vi "FlexMag - 23-03-2023.vi"() -> ()   [LabVIEW 2018] (continued)
                            tunnel: [w16037 TRUE ("CH1_Trns_BP_Left_DO")] -> w16029
                            frame False {
                              n10680 = local read "CH2_TGV_Control_DI"() -> (w16038:bool)
                              n10681 = case shown="False" w16038 {
                                tunnel: [FALSE ("CH1_Trns_BP_Left_DO") TRUE ("CH1_Trns_BP_Left_DO")] -> w16037
                                frame False {
                                n10682 = Wait Until Next ms Multiple(millisecond multiple=u32 200) -> ()  [unwired: 1 out]
                                n10683 = local write "CH2_TGV_Control_DO"(TRUE ("CH1_Trns_BP_Left_DO")) -> ()
                                }
                                frame True {
                                }
                              }
                            }
                            frame True {
                            }
                          }
                          n10684 = local read "ch2-1 transfer"() -> (w16036:bool)
                          n10685 = local read "ABORT"() -> (w16035:bool)
                          n10686 = Not(x=w16036) -> (.not. x?=w16034:bool)
                          n10687 = Compound Arithmetic op=OR(w16029, w16035, w16034) -> (w16033:bool)
                        }
                      }
                      frame True {
                      }
                    }
                  }
                }
              }
              frame #12 {
                n10688 = local read "ch2-1 transfer"() -> (w16046:bool)
                n10689 = case shown="True" w16046 {
                  frame False {
                  }
                  frame True {
                    n10690 = local read "ABORT"() -> (w16047:bool)
                    n10691 = case shown="False" w16047 {
                      frame False {
                        w16048 = TRUE ("CH2_Right_Limit_DO")
                        n10692 = local write "trns 2-1 led 5"(TRUE ("trns 1-2 led 1")) -> ()
                        n10693 = Wait (ms)(milliseconds to wait=u32 100) -> ()  [unwired: 1 out]
                        n10694 = local write "CH2_Right_Limit_DO"(w16048) -> ()
                        n10695 = local write "CH2_Right_Slow_DO"(w16048) -> ()
                        n10696 = local write "CH2_Left_Slow_DO"(w16048) -> ()
                        n10697 = local write "CH2_Left_Limit_DO"(w16048) -> ()
                      }
                      frame True {
                      }
                    }
                  }
                }
              }
              frame #13 {
                n10698 = local read "ch2-1 transfer"() -> (w16051:bool)
                n10699 = case shown="True" w16051 {
                  frame False {
                  }
                  frame True {
                    n10700 = local read "ABORT"() -> (w16052:bool)
                    n10701 = case shown="False" w16052 {
                      frame False {
                        n10702 = while {
                          i -> [w16057]
                          stop <- w16058 stop-if-true
                          n10703 = local read "CH3_Trns_Interlock_DI"() -> (w16053:bool)
                          n10704 = Greater Or Equal?(x=w16057, y=100) -> (x >= y?=w16055:bool)
                          n10705 = case shown="True" w16055 {
                            frame False {
                            }
                            frame True {
                              n10706 = local write "Warning Message"("Transfer process canceled!\nCH3 Interlock problem" ("Warning Message")) -> ()
                              n10707 = local write "trns error"(TRUE ("TRNS error")) -> ()
                            }
                          }
                          n10708 = case shown="False" w16053 {
                            tunnel: [w16062 TRUE ("CH1_Trns_BP_Left_DO")] -> w16054
                            frame False {
                              n10709 = local read "CH3_TGV_Control_DI"() -> (w16063:bool)
                              n10710 = case shown="False" w16063 {
                                tunnel: [FALSE ("CH1_Trns_BP_Left_DO") TRUE ("CH1_Trns_BP_Left_DO")] -> w16062
                                frame False {
                                n10711 = Wait Until Next ms Multiple(millisecond multiple=u32 200) -> ()  [unwired: 1 out]
                                n10712 = local write "CH3_TGV_Control_DO"(TRUE ("CH1_Trns_BP_Left_DO")) -> ()
                                }
                                frame True {
                                }
                              }
                            }
                            frame True {
                            }
                          }
                          n10713 = local read "ch2-1 transfer"() -> (w16061:bool)
                          n10714 = local read "ABORT"() -> (w16060:bool)
                          n10715 = Not(x=w16061) -> (.not. x?=w16059:bool)
                          n10716 = Compound Arithmetic op=OR(w16054, w16060, w16059) -> (w16058:bool)
                        }
                      }
                      frame True {
                      }
                    }
                  }
                }
              }
              frame #14 {
                n10717 = local read "ch2-1 transfer"() -> (w16071:bool)
                n10718 = case shown="True" w16071 {
                  frame False {
                  }
                  frame True {
                    n10719 = local read "ABORT"() -> (w16072:bool)
                    n10720 = case shown="False" w16072 {
                      frame False {
                        n10721 = local write "trns 2-1 led 6"(TRUE ("trns 1-2 led 1")) -> ()
                        n10722 = Wait (ms)(milliseconds to wait=u32 100) -> ()  [unwired: 1 out]
                      }
                      frame True {
                      }
                    }
                  }
                }
              }
              frame #15 {
                n10723 = local read "ch2-1 transfer"() -> (w16075:bool)
                n10724 = case shown="True" w16075 {
                  frame False {
                  }
                  frame True {
                    n10725 = local read "ABORT"() -> (w16076:bool)
                    n10726 = case shown="False" w16076 {
                      frame False {
                        n10727 = while {
                          i -> [w16081]
                          stop <- w16082 stop-if-true
                          n10728 = local read "CH4_Trns_Interlock_DI"() -> (w16077:bool)
                          n10729 = Greater Or Equal?(x=w16081, y=100) -> (x >= y?=w16079:bool)
                          n10730 = case shown="True" w16079 {
                            frame False {
                            }
                            frame True {
                              n10731 = local write "Warning Message"("Transfer process canceled!\nCH4 Interlock problem" ("Warning Message")) -> ()
                              n10732 = local write "trns error"(TRUE ("TRNS error")) -> ()
                            }
                          }
                          n10733 = case shown="False" w16077 {
                            tunnel: [w16086 TRUE ("CH1_Trns_BP_Left_DO")] -> w16078
                            frame False {
                              n10734 = local read "CH4_TGV_Control_DI"() -> (w16087:bool)
                              n10735 = case shown="False" w16087 {
                                tunnel: [FALSE ("CH1_Trns_BP_Left_DO") TRUE ("CH1_Trns_BP_Left_DO")] -> w16086
                                frame False {
                                n10736 = Wait Until Next ms Multiple(millisecond multiple=u32 200) -> ()  [unwired: 1 out]
                                n10737 = local write "CH4_TGV_Control_DO"(TRUE ("CH1_Trns_BP_Left_DO")) -> ()
                                }
                                frame True {
                                }
                              }
                            }
                            frame True {
                            }
                          }
                          n10738 = local read "ch2-1 transfer"() -> (w16085:bool)
                          n10739 = local read "ABORT"() -> (w16084:bool)
                          n10740 = Not(x=w16085) -> (.not. x?=w16083:bool)
                          n10741 = Compound Arithmetic op=OR(w16078, w16084, w16083) -> (w16082:bool)
                        }
                      }
                      frame True {
                      }
                    }
                  }
                }
              }
              frame #16 {
                n10742 = local read "ch2-1 transfer"() -> (w16095:bool)
                n10743 = case shown="True" w16095 {
                  frame False {
                  }
                  frame True {
                    n10744 = local read "ABORT"() -> (w16096:bool)
                    n10745 = case shown="False" w16096 {
                      frame False {
                        n10746 = local write "trns 2-1 led 7"(TRUE ("trns 1-2 led 1")) -> ()
                        n10747 = Wait (ms)(milliseconds to wait=u32 100) -> ()  [unwired: 1 out]
                      }
                      frame True {
                      }
                    }
                  }
                }
              }
              frame #17 {
                n10748 = local read "ch2-1 transfer"() -> (w16099:bool)
                n10749 = case shown="True" w16099 {
                  frame False {
                  }
                  frame True {
                    n10750 = local read "ABORT"() -> (w16100:bool)
                    n10751 = case shown="False" w16100 {
                      frame False {
                        n10752 = while {
                          i -> [w16104]
                          stop <- w16105 stop-if-true
                          n10753 = Greater Or Equal?(x=w16104, y=100) -> (x >= y?=w16102:bool)
                          n10754 = case shown="True" w16102 {
                            frame False {
                            }
                            frame True {
                              n10755 = local write "Warning Message"("Transfer process canceled!\nRight Slow Sensor problem" ("Warning Message")) -> ()
                              n10756 = local write "trns error"(TRUE ("TRNS error")) -> ()
                            }
                          }
                          n10757 = disable-structure shown="Enabled" {
                            disable-tunnel: [w16110 w16115] -> w16101
                            frame Disabled {
                              n10758 = local read "Cnt_Right_Slow DI"() -> (w16109:bool)
                              n10759 = case shown="False" w16109 {
                                tunnel: [FALSE ("CH1_Trns_BP_Left_DO") TRUE ("CH1_Trns_BP_Left_DO")] -> w16110
                                frame False {
                                n10760 = Wait Until Next ms Multiple(millisecond multiple=u32 200) -> ()  [unwired: 1 out]
                                n10761 = local write "Cnt_Right_Slow DO"(TRUE ("CH1_Trns_BP_Left_DO")) -> ()
                                }
                                frame True {
                                }
                              }
                            }
                            frame Enabled {
                              n10762 = local read "CH2_Right_Slow_DI"() -> (w16116:bool)
                              n10763 = case shown="True" w16116 {
                                tunnel: [TRUE FALSE] -> w16115
                                frame False {
                                }
                                frame True {
                                n10764 = Wait Until Next ms Multiple(millisecond multiple=u32 200) -> ()  [unwired: 1 out]
                                n10765 = local write "CH2_Right_Slow_DO"(TRUE ("CH2_Right_Limit_DO")) -> ()
                                }
                              }
                            }
                          }
                          n10766 = local read "ch2-1 transfer"() -> (w16108:bool)
                          n10767 = local read "ABORT"() -> (w16107:bool)
                          n10768 = Not(x=w16108) -> (.not. x?=w16106:bool)
                          n10769 = Compound Arithmetic op=OR(w16101, w16107, w16106) -> (w16105:bool)
                        }
                      }
                      frame True {
                      }
                    }
                  }
                }
              }
              frame #18 {
                n10770 = local read "ch2-1 transfer"() -> (w16123:bool)
                n10771 = case shown="True" w16123 {
                  frame False {
                  }
                  frame True {
                    n10772 = local read "ABORT"() -> (w16124:bool)
                    n10773 = case shown="False" w16124 {
                      frame False {
                        n10774 = local write "trns 2-1 led 8"(TRUE ("trns 1-2 led 1")) -> ()
                        n10775 = Wait (ms)(milliseconds to wait=u32 100) -> ()  [unwired: 1 out]
                      }
                      frame True {
                      }
                    }
                  }
                }
              }
              frame #19 {
                n10776 = local read "ch2-1 transfer"() -> (w16127:bool)
                n10777 = case shown="True" w16127 {
                  frame False {
                  }
                  frame True {
                    n10778 = local read "ABORT"() -> (w16128:bool)
                    n10779 = case shown="False" w16128 {
                      frame False {
                        n10780 = while {
                          i -> [w16132]
                          stop <- w16133 stop-if-true
                          n10781 = Greater Or Equal?(x=w16132, y=100) -> (x >= y?=w16130:bool)
                          n10782 = case shown="True" w16130 {
                            frame False {
                            }
                            frame True {
                              n10783 = local write "Warning Message"("Transfer process canceled!\nRight Limit Sensor problem" ("Warning Message")) -> ()
                              n10784 = local write "trns error"(TRUE ("TRNS error")) -> ()
                            }
                          }
                          n10785 = disable-structure shown="Enabled" {
                            disable-tunnel: [w16138 w16143] -> w16129
                            frame Disabled {
                              n10786 = local read "Cnt_Right_Limit DI"() -> (w16137:bool)
                              n10787 = case shown="False" w16137 {
                                tunnel: [FALSE ("CH1_Trns_BP_Left_DO") TRUE ("CH1_Trns_BP_Left_DO")] -> w16138
                                frame False {
                                n10788 = Wait Until Next ms Multiple(millisecond multiple=u32 200) -> ()  [unwired: 1 out]
                                n10789 = local write "Cnt_Right_Limit DO"(TRUE ("CH1_Trns_BP_Left_DO")) -> ()
                                }
                                frame True {
                                }
                              }
                            }
                            frame Enabled {
                              n10790 = local read "CH2_Right_Limit_DI"() -> (w16144:bool)
                              n10791 = case shown="True" w16144 {
                                tunnel: [TRUE FALSE] -> w16143
                                frame False {
                                }
                                frame True {
                                n10792 = Wait Until Next ms Multiple(millisecond multiple=u32 200) -> ()  [unwired: 1 out]
                                n10793 = local write "CH2_Right_Limit_DO"(TRUE ("CH2_Right_Limit_DO")) -> ()
                                }
                              }
                            }
                          }
                          n10794 = local read "ch2-1 transfer"() -> (w16136:bool)
                          n10795 = local read "ABORT"() -> (w16135:bool)
                          n10796 = Not(x=w16136) -> (.not. x?=w16134:bool)
                          n10797 = Compound Arithmetic op=OR(w16129, w16135, w16134) -> (w16133:bool)
                        }
                      }
                      frame True {
                      }
                    }
                  }
                }
              }
              frame #20 {
                n10798 = local read "ch2-1 transfer"() -> (w16151:bool)
                n10799 = case shown="True" w16151 {
                  frame False {
                  }
                  frame True {
                    n10800 = local read "ABORT"() -> (w16152:bool)
                    n10801 = case shown="False" w16152 {
                      frame False {
                        n10802 = local write "trns 2-1 led 9"(TRUE ("trns 1-2 led 1")) -> ()
                        n10803 = Wait (ms)(milliseconds to wait=u32 100) -> ()  [unwired: 1 out]
                      }
                      frame True {
                      }
                    }
                  }
                }
              }
              frame #21 {
                n10804 = local read "ch2-1 transfer"() -> (w16155:bool)
                n10805 = case shown="True" w16155 {
                  frame False {
                  }
                  frame True {
                    n10806 = local read "ABORT"() -> (w16156:bool)
                    n10807 = case shown="False" w16156 {
                      frame False {
                        n10808 = while {
                          i -> [w16160]
                          stop <- w16161 stop-if-true
                          n10809 = Greater Or Equal?(x=w16160, y=100) -> (x >= y?=w16158:bool)
                          n10810 = case shown="True" w16158 {
                            frame False {
                            }
                            frame True {
                              n10811 = local write "Warning Message"("Transfer process canceled!\nLeft Slow Sensor problem" ("Warning Message")) -> ()
                              n10812 = local write "trns error"(TRUE ("TRNS error")) -> ()
                            }
                          }
                          n10813 = disable-structure shown="Enabled" {
                            disable-tunnel: [w16166 w16171] -> w16157
                            frame Disabled {
                              n10814 = local read "Cnt_Left_Slow DI"() -> (w16165:bool)
                              n10815 = case shown="False" w16165 {
                                tunnel: [FALSE ("CH1_Trns_BP_Left_DO") TRUE ("CH1_Trns_BP_Left_DO")] -> w16166
                                frame False {
                                n10816 = Wait Until Next ms Multiple(millisecond multiple=u32 200) -> ()  [unwired: 1 out]
                                n10817 = local write "Cnt_Left_Slow DO"(TRUE ("CH1_Trns_BP_Left_DO")) -> ()
                                }
                                frame True {
                                }
                              }
                            }
                            frame Enabled {
                              n10818 = local read "CH2_Left_Slow_DI"() -> (w16172:bool)
                              n10819 = case shown="True" w16172 {
                                tunnel: [TRUE FALSE] -> w16171
                                frame False {
                                }
                                frame True {
                                n10820 = Wait Until Next ms Multiple(millisecond multiple=u32 200) -> ()  [unwired: 1 out]
                                n10821 = local write "CH2_Left_Slow_DO"(TRUE ("CH2_Right_Limit_DO")) -> ()
                                }
                              }
                            }
                          }
                          n10822 = local read "ch2-1 transfer"() -> (w16164:bool)
                          n10823 = local read "ABORT"() -> (w16163:bool)
                          n10824 = Not(x=w16164) -> (.not. x?=w16162:bool)
                          n10825 = Compound Arithmetic op=OR(w16157, w16163, w16162) -> (w16161:bool)
                        }
                      }
                      frame True {
                      }
                    }
                  }
                }
              }
              frame #22 {
                n10826 = local read "ch2-1 transfer"() -> (w16179:bool)
                n10827 = case shown="True" w16179 {
                  frame False {
                  }
                  frame True {
                    n10828 = local read "ABORT"() -> (w16180:bool)
                    n10829 = case shown="False" w16180 {
                      frame False {
                        n10830 = local write "trns 2-1 led 10"(TRUE ("trns 1-2 led 1")) -> ()
                        n10831 = Wait (ms)(milliseconds to wait=u32 100) -> ()  [unwired: 1 out]
                      }
                      frame True {
                      }
                    }
                  }
                }
              }
              frame #23 {
                n10832 = local read "ch2-1 transfer"() -> (w16183:bool)
                n10833 = case shown="True" w16183 {
                  frame False {
                  }
                  frame True {
                    n10834 = local read "ABORT"() -> (w16184:bool)
                    n10835 = case shown="False" w16184 {
                      frame False {
                        n10836 = while {
                          i -> [w16188]
                          stop <- w16189 stop-if-true
                          n10837 = Greater Or Equal?(x=w16188, y=100) -> (x >= y?=w16186:bool)
                          n10838 = case shown="True" w16186 {
                            frame False {
                            }
                            frame True {
                              n10839 = local write "Warning Message"("Transfer process canceled!\nLeft Limit Sensor problem" ("Warning Message")) -> ()
                              n10840 = local write "trns error"(TRUE ("TRNS error")) -> ()
                            }
                          }
                          n10841 = disable-structure shown="Enabled" {
                            disable-tunnel: [w16194 w16199] -> w16185
                            frame Disabled {
                              n10842 = local read "Cnt_Left_Limit DI"() -> (w16193:bool)
                              n10843 = case shown="False" w16193 {
                                tunnel: [FALSE ("CH1_Trns_BP_Left_DO") TRUE ("CH1_Trns_BP_Left_DO")] -> w16194
                                frame False {
                                n10844 = Wait Until Next ms Multiple(millisecond multiple=u32 200) -> ()  [unwired: 1 out]
                                n10845 = local write "Cnt_Left_Limit DO"(TRUE ("CH1_Trns_BP_Left_DO")) -> ()
                                }
                                frame True {
                                }
                              }
                            }
                            frame Enabled {
                              n10846 = local read "CH2_Left_Limit_DI"() -> (w16200:bool)
                              n10847 = case shown="True" w16200 {
                                tunnel: [TRUE FALSE] -> w16199
                                frame False {
                                }
                                frame True {
                                n10848 = Wait Until Next ms Multiple(millisecond multiple=u32 200) -> ()  [unwired: 1 out]
                                n10849 = local write "CH2_Left_Limit_DO"(TRUE ("CH2_Right_Limit_DO")) -> ()
                                }
                              }
                            }
                          }
                          n10850 = local read "ch2-1 transfer"() -> (w16192:bool)
                          n10851 = local read "ABORT"() -> (w16191:bool)
                          n10852 = Not(x=w16192) -> (.not. x?=w16190:bool)
                          n10853 = Compound Arithmetic op=OR(w16185, w16191, w16190) -> (w16189:bool)
                        }
                      }
                      frame True {
                      }
                    }
                  }
                }
              }
              frame #24 {
                n10854 = local read "ch2-1 transfer"() -> (w16207:bool)
                n10855 = case shown="True" w16207 {
                  frame False {
                  }
                  frame True {
                    n10856 = local read "ABORT"() -> (w16208:bool)
                    n10857 = case shown="False" w16208 {
                      frame False {
                        n10858 = local write "trns 2-1 led 11"(TRUE ("trns 1-2 led 1")) -> ()
                        n10859 = Wait (ms)(milliseconds to wait=u32 100) -> ()  [unwired: 1 out]
                      }
                      frame True {
                      }
                    }
                  }
                }
              }
              frame #25 {
                n10860 = local read "ch2-1 transfer"() -> (w16211:bool)
                n10861 = case shown="True" w16211 {
                  frame False {
                  }
                  frame True {
                    n10862 = local read "ABORT"() -> (w16212:bool)
                    n10863 = case shown="False" w16212 {
                      frame False {
                        w16213 = FALSE ("CH1_Right_Limit_DO")
                        n10864 = local write "CH1_Right_Limit_DO"(w16213) -> ()
                        n10865 = local write "CH1_Right_Slow_DO"(w16213) -> ()
                        n10866 = Wait (ms)(milliseconds to wait=u32 2000) -> ()  [unwired: 1 out]
                      }
                      frame True {
                      }
                    }
                  }
                }
              }
              frame #26 {
                n10867 = local read "ch2-1 transfer"() -> (w16215:bool)
                n10868 = case shown="True" w16215 {
                  frame False {
                  }
                  frame True {
                    n10869 = local read "ABORT"() -> (w16216:bool)
                    n10870 = case shown="False" w16216 {
                      frame False {
                        n10871 = while {
                          i -> [w16221]
                          stop <- w16222 stop-if-true
                          n10872 = Greater Or Equal?(x=w16221, y=100) -> (x >= y?=w16219:bool)
                          n10873 = case shown="True" w16219 {
                            frame False {
                            }
                            frame True {
                              n10874 = local write "Warning Message"("Transfer process canceled!\nCassette Servo Direction problem" ("Warning Message")) -> ()
                              n10875 = local write "trns error"(TRUE ("TRNS error")) -> ()
                            }
                          }
                          n10876 = local read "Casette_Servo_Left_Direction DI"() -> (w16217:bool)
                          n10877 = case shown="True" w16217 {
                            tunnel: [TRUE ("CH1_Trns_BP_Left_DO") FALSE ("CH1_Trns_BP_Left_DO")] -> w16218
                            frame False {
                            }
                            frame True {
                              n10878 = local write "Casette_Servo_Left_Direction DO"(FALSE ("CH1_Trns_BP_Left_DO")) -> ()
                              n10879 = Wait Until Next ms Multiple(millisecond multiple=u32 200) -> ()  [unwired: 1 out]
                            }
                          }
                          n10880 = local read "ch2-1 transfer"() -> (w16225:bool)
                          n10881 = local read "ABORT"() -> (w16224:bool)
                          n10882 = Not(x=w16225) -> (.not. x?=w16223:bool)
                          n10883 = Compound Arithmetic op=OR(w16218, w16224, w16223) -> (w16222:bool)
                        }
                      }
                      frame True {
                      }
                    }
                  }
                }
              }
              frame #27 {
                n10884 = local read "ch2-1 transfer"() -> (w16232:bool)
                n10885 = case shown="True" w16232 {
                  frame False {
                  }
                  frame True {
                    n10886 = local read "ABORT"() -> (w16233:bool)
                    n10887 = case shown="False" w16233 {
                      frame False {
                        n10888 = local write "trns 2-1 led 12"(TRUE ("trns 1-2 led 1")) -> ()
                        n10889 = Wait (ms)(milliseconds to wait=u32 100) -> ()  [unwired: 1 out]
                      }
                      frame True {
                      }
                    }
                  }
                }
              }
              frame #28 {
                n10890 = local read "ch2-1 transfer"() -> (w16236:bool)
                n10891 = case shown="True" w16236 {
                  frame False {
                  }
                  frame True {
                    n10892 = local read "ABORT"() -> (w16237:bool)
                    n10893 = case shown="False" w16237 {
                      frame False {
                        n10894 = stacked-sequence {
                          frame #0 {
                            n10895 = local read "Cst_Speed_High"() -> (w16238:dbl)
                            n10896 = Wait (ms)(milliseconds to wait=u32 100) -> ()  [unwired: 1 out]
                            n10897 = local write "Cassette_Servo_Speed AO"(w16238) -> ()
                          }
                          frame #1 {
                            n10898 = Wait (ms)(milliseconds to wait=u32 200) -> ()  [unwired: 1 out]
                          }
                          frame #2 {
                            n10899 = local write "Cassette_Servo_Speed Set"(TRUE ("Cassette_Servo_Speed Set")) -> ()
                          }
                          frame #3 {
                            n10900 = Wait (ms)(milliseconds to wait=u32 300) -> ()  [unwired: 1 out]
                          }
                        }
                      }
                      frame True {
                      }
                    }
                  }
                }
              }
              frame #29 {
                n10901 = local read "ch2-1 transfer"() -> (w16243:bool)
                n10902 = case shown="True" w16243 {
                  frame False {
                  }
                  frame True {
                    n10903 = local read "ABORT"() -> (w16244:bool)
                    n10904 = case shown="False" w16244 {
                      frame False {
                        n10905 = local write "trns 2-1 led 13"(TRUE ("trns 1-2 led 1")) -> ()
                        n10906 = Wait (ms)(milliseconds to wait=u32 100) -> ()  [unwired: 1 out]
                      }
                      frame True {
                      }
                    }
                  }
                }
              }
              frame #30 {
                n10907 = local read "ch2-1 transfer"() -> (w16247:bool)
                n10908 = case shown="True" w16247 {
                  frame False {
                  }
                  frame True {
                    n10909 = local read "ABORT"() -> (w16248:bool)
                    n10910 = case shown="False" w16248 {
                      frame False {
                        n10911 = while {
                          i -> [w16253]
                          stop <- w16254 stop-if-true
                          n10912 = Greater Or Equal?(x=w16253, y=100) -> (x >= y?=w16251:bool)
                          n10913 = case shown="True" w16251 {
                            frame False {
                            }
                            frame True {
                              n10914 = local write "Warning Message"("Transfer process canceled!\nCassette Servo Start problem" ("Warning Message")) -> ()
                              n10915 = local write "trns error"(TRUE ("TRNS error")) -> ()
                            }
                          }
                          n10916 = local read "Casette_Servo_Start/Stop DI"() -> (w16249:bool)
                          n10917 = case shown="False" w16249 {
                            tunnel: [FALSE ("CH1_Trns_BP_Left_DO") TRUE ("CH1_Trns_BP_Left_DO")] -> w16250
                            frame False {
                              n10918 = local write "Casette_Servo_Start/Stop DO"(TRUE ("CH1_Trns_BP_Left_DO")) -> ()
                              n10919 = Wait Until Next ms Multiple(millisecond multiple=u32 200) -> ()  [unwired: 1 out]
                            }
                            frame True {
                            }
                          }
                          n10920 = local read "ch2-1 transfer"() -> (w16257:bool)
                          n10921 = local read "ABORT"() -> (w16256:bool)
                          n10922 = Not(x=w16257) -> (.not. x?=w16255:bool)
                          n10923 = Compound Arithmetic op=OR(w16250, w16256, w16255) -> (w16254:bool)
                        }
                      }
                      frame True {
                      }
                    }
                  }
                }
              }
              frame #31 {
                n10924 = local read "ch2-1 transfer"() -> (w16264:bool)
                n10925 = case shown="True" w16264 {
                  frame False {
                  }
                  frame True {
                    n10926 = local read "ABORT"() -> (w16265:bool)
                    n10927 = case shown="False" w16265 {
                      frame False {
                        n10928 = local write "trns 2-1 led 14"(TRUE ("trns 1-2 led 1")) -> ()
                        n10929 = Wait (ms)(milliseconds to wait=u32 100) -> ()  [unwired: 1 out]
                      }
                      frame True {
                      }
                    }
                  }
                }
              }
              frame #32 {
                n10930 = local read "ch2-1 transfer"() -> (w16268:bool)
                n10931 = case shown="True" w16268 {
                  frame False {
                  }
                  frame True {
                    n10932 = local read "ABORT"() -> (w16269:bool)
                    n10933 = case shown="False" w16269 {
                      frame False {
                        n10934 = disable-structure shown="Disabled" {
                          frame Disabled {
                            n10935 = stacked-sequence {
                              frame #0 {
                                n10936 = while {
                                i -> [w16276]
                                stop <- w16277 stop-if-true
                                n10937 = Greater Or Equal?(x=w16276, y=1500) -> (x >= y?=w16274:bool)
                                n10938 = case shown="True" w16274 {
                                frame False {
                                }
                                frame True {
                                n10939 = local write "Warning Message"("Transfer process canceled!\nCounter problem" ("Warning Message")) -> ()
                                n10940 = local write "trns error"(TRUE ("TRNS error")) -> ()
                                }
                                }
                                n10941 = local read "Counter Read Data"() -> (w16272:i16)
                                n10942 = Less Or Equal?(x=w16272, y=i16 800) -> (x <= y?=w16270:bool)
                                n10943 = case shown="False" w16270 {
                                tunnel: [FALSE ("CH1_Trns_BP_Left_DO") TRUE ("CH1_Trns_BP_Left_DO")] -> w16273
                                frame False {
                                n10944 = Wait Until Next ms Multiple(millisecond multiple=u32 200) -> ()  [unwired: 1 out]
                                }
                                frame True {
                                }
                                }
                                n10945 = local read "ch2-1 transfer"() -> (w16280:bool)
                                n10946 = local read "ABORT"() -> (w16279:bool)
                                n10947 = Not(x=w16280) -> (.not. x?=w16278:bool)
                                n10948 = Compound Arithmetic op=OR(w16273, w16279, w16278) -> (w16277:bool)
                                }
                              }
                              frame #1 {
                                n10949 = while {
                                i -> [w16290]
                                stop <- w16291 stop-if-true
                                n10950 = Greater Or Equal?(x=w16290, y=100) -> (x >= y?=w16288:bool)
                                n10951 = case shown="True" w16288 {
                                frame False {
                                }
                                frame True {
                                n10952 = local write "Warning Message"("Transfer process canceled!\nRight Slow Sensor problem" ("Warning Message")) -> ()
                                n10953 = local write "trns error"(TRUE ("TRNS error")) -> ()
                                }
                                }
                                n10954 = local read "Cnt_Right_Slow DI"() -> (w16286:bool)
                                n10955 = case shown="True" w16286 {
                                tunnel: [TRUE ("CH1_Trns_BP_Left_DO") FALSE ("CH1_Trns_BP_Left_DO")] -> w16287
                                frame False {
                                }
                                frame True {
                                n10956 = Wait Until Next ms Multiple(millisecond multiple=u32 200) -> ()  [unwired: 1 out]
                                n10957 = local write "Cnt_Right_Slow DO"(FALSE ("TRNS error")) -> ()
                                }
                                }
                                n10958 = local read "ch2-1 transfer"() -> (w16294:bool)
                                n10959 = local read "ABORT"() -> (w16293:bool)
                                n10960 = Not(x=w16294) -> (.not. x?=w16292:bool)
                                n10961 = Compound Arithmetic op=OR(w16287, w16293, w16292) -> (w16291:bool)
                                }
                              }
                              frame #2 {
                                n10962 = while {
                                i -> [w16305]
                                stop <- w16306 stop-if-true
                                n10963 = Greater Or Equal?(x=w16305, y=100) -> (x >= y?=w16303:bool)
                                n10964 = case shown="True" w16303 {
                                frame False {
                                }
                                frame True {
                                n10965 = local write "Warning Message"("Transfer process canceled!\nRight Limit Sensor problem" ("Warning Message")) -> ()
                                n10966 = local write "trns error"(TRUE ("TRNS error")) -> ()
                                }
                                }
                                n10967 = local read "Cnt_Right_Limit DI"() -> (w16301:bool)
                                n10968 = case shown="True" w16301 {
                                tunnel: [TRUE ("CH1_Trns_BP_Left_DO") FALSE ("CH1_Trns_BP_Left_DO")] -> w16302
                                frame False {
                                }
                                frame True {
                                n10969 = Wait Until Next ms Multiple(millisecond multiple=u32 200) -> ()  [unwired: 1 out]
                                n10970 = local write "Cnt_Right_Limit DO"(FALSE ("TRNS error")) -> ()
                                }
                                }
                                n10971 = local read "ch2-1 transfer"() -> (w16309:bool)
                                n10972 = local read "ABORT"() -> (w16308:bool)
                                n10973 = Not(x=w16309) -> (.not. x?=w16307:bool)
                                n10974 = Compound Arithmetic op=OR(w16302, w16308, w16307) -> (w16306:bool)
                                }
                              }
                            }
                          }
                          frame Enabled {
                          }
                        }
                      }
                      frame True {
                      }
                    }
                  }
                }
              }
              frame #33 {
                n10975 = local read "ch2-1 transfer"() -> (w16316:bool)
                n10976 = case shown="True" w16316 {
                  frame False {
                  }
                  frame True {
                    n10977 = local read "ABORT"() -> (w16317:bool)
                    n10978 = case shown="False" w16317 {
                      frame False {
                        n10979 = local write "trns 2-1 led 15"(TRUE ("trns 1-2 led 1")) -> ()
                        n10980 = Wait (ms)(milliseconds to wait=u32 100) -> ()  [unwired: 1 out]
                      }
                      frame True {
                      }
                    }
                  }
                }
              }
              frame #34 {
                n10981 = local read "ch2-1 transfer"() -> (w16320:bool)
                n10982 = case shown="True" w16320 {
                  frame False {
                  }
                  frame True {
                    n10983 = local read "ABORT"() -> (w16321:bool)
                    n10984 = case shown="False" w16321 {
                      frame False {
                        n10985 = stacked-sequence {
                          frame #0 {
                            n10986 = while {
                              i -> [w16326]
                              stop <- w16327 stop-if-true
                              n10987 = Greater Or Equal?(x=w16326, y=1500) -> (x >= y?=w16324:bool)
                              n10988 = case shown="True" w16324 {
                                frame False {
                                }
                                frame True {
                                n10989 = local write "Warning Message"("Transfer process canceled!\nCH1 Right Slow Sensor problem" ("Warning Message")) -> ()
                                n10990 = local write "trns error"(TRUE ("TRNS error")) -> ()
                                }
                              }
                              n10991 = local read "CH1_Right_Slow_DI"() -> (w16322:bool)
                              n10992 = case shown="True" w16322 {
                                tunnel: [FALSE ("CH1_Trns_BP_Left_DO") TRUE ("CH1_Trns_BP_Left_DO")] -> w16323
                                frame False {
                                n10993 = Wait Until Next ms Multiple(millisecond multiple=u32 200) -> ()  [unwired: 1 out]
                                }
                                frame True {
                                }
                              }
                              n10994 = local read "ch2-1 transfer"() -> (w16330:bool)
                              n10995 = local read "ABORT"() -> (w16329:bool)
                              n10996 = Not(x=w16330) -> (.not. x?=w16328:bool)
                              n10997 = Compound Arithmetic op=OR(w16323, w16329, w16328) -> (w16327:bool)
                            }
                          }
                          frame #1 {
                            n10998 = flat-sequence {
                              frame #0 {
                                n10999 = local read "Cst_Speed_Low"() -> (w16336:dbl)
                                n11000 = local write "Cassette_Servo_Speed AO"(w16336) -> ()
                                n11001 = Wait (ms)(milliseconds to wait=u32 100) -> ()  [unwired: 1 out]
                              }
                              frame #1 {
                                n11002 = local write "Cassette_Servo_Speed Set"(TRUE ("Cassette_Servo_Speed Set")) -> ()
                              }
                              frame #2 {
                                n11003 = Wait (ms)(milliseconds to wait=u32 100) -> ()  [unwired: 1 out]
                              }
                            }
                          }
                          frame #2 {
                            n11004 = while {
                              i -> [w16343]
                              stop <- w16344 stop-if-true
                              n11005 = Greater Or Equal?(x=w16343, y=100) -> (x >= y?=w16341:bool)
                              n11006 = case shown="True" w16341 {
                                frame False {
                                }
                                frame True {
                                n11007 = local write "Warning Message"("Transfer process canceled!\nRight Slow Sensor problem" ("Warning Message")) -> ()
                                n11008 = local write "trns error"(TRUE ("TRNS error")) -> ()
                                }
                              }
                              n11009 = disable-structure shown="Enabled" {
                                disable-tunnel: [w16349 w16354] -> w16340
                                frame Disabled {
                                n11010 = local read "Cnt_Right_Slow DI"() -> (w16348:bool)
                                n11011 = case shown="False" w16348 {
                                tunnel: [FALSE ("CH1_Trns_BP_Left_DO") TRUE ("CH1_Trns_BP_Left_DO")] -> w16349
                                frame False {
                                n11012 = Wait Until Next ms Multiple(millisecond multiple=u32 200) -> ()  [unwired: 1 out]
                                n11013 = local write "Cnt_Right_Slow DO"(TRUE ("TRNS error")) -> ()
                                }
                                frame True {
                                }
                                }
                                }
                                frame Enabled {
                                n11014 = local read "CH1_Right_Slow_DI"() -> (w16355:bool)
                                n11015 = case shown="True" w16355 {
                                tunnel: [TRUE FALSE] -> w16354
                                frame False {
                                }
                                frame True {
                                n11016 = Wait Until Next ms Multiple(millisecond multiple=u32 200) -> ()  [unwired: 1 out]
                                n11017 = local write "CH1_Right_Slow_DO"(TRUE ("CH2_Right_Limit_DO")) -> ()
                                }
                                }
                                }
                              }
                              n11018 = local read "ch2-1 transfer"() -> (w16347:bool)
                              n11019 = local read "ABORT"() -> (w16346:bool)
                              n11020 = Not(x=w16347) -> (.not. x?=w16345:bool)
                              n11021 = Compound Arithmetic op=OR(w16340, w16346, w16345) -> (w16344:bool)
                            }
                          }
                        }
                      }
                      frame True {
                      }
                    }
                  }
                }
              }
              frame #35 {
                n11022 = local read "ch2-1 transfer"() -> (w16362:bool)
                n11023 = case shown="True" w16362 {
                  frame False {
                  }
                  frame True {
                    n11024 = local read "ABORT"() -> (w16363:bool)
                    n11025 = case shown="False" w16363 {
                      frame False {
                        n11026 = local write "trns 2-1 led 16"(TRUE ("trns 1-2 led 1")) -> ()
                        n11027 = Wait (ms)(milliseconds to wait=u32 100) -> ()  [unwired: 1 out]
                      }
                      frame True {
                      }
                    }
                  }
                }
              }
              frame #36 {
                n11028 = local read "ch2-1 transfer"() -> (w16366:bool)
                n11029 = case shown="True" w16366 {
                  frame False {
                  }
                  frame True {
                    n11030 = local read "ABORT"() -> (w16367:bool)
                    n11031 = case shown="False" w16367 {
                      frame False {
                        n11032 = stacked-sequence {
                          frame #0 {
                            n11033 = while {
                              i -> [w16372]
                              stop <- w16373 stop-if-true
                              n11034 = Greater Or Equal?(x=w16372, y=600) -> (x >= y?=w16370:bool)
                              n11035 = case shown="True" w16370 {
                                frame False {
                                }
                                frame True {
                                n11036 = local write "Warning Message"("Transfer process canceled!\nCH1 Right Limit Sensor problem" ("Warning Message")) -> ()
                                n11037 = local write "trns error"(TRUE ("TRNS error")) -> ()
                                }
                              }
                              n11038 = local read "CH1_Right_Limit_DI"() -> (w16368:bool)
                              n11039 = case shown="True" w16368 {
                                tunnel: [FALSE ("CH1_Trns_BP_Left_DO") TRUE ("CH1_Trns_BP_Left_DO")] -> w16369
                                frame False {
                                n11040 = Wait Until Next ms Multiple(millisecond multiple=u32 200) -> ()  [unwired: 1 out]
                                }
                                frame True {
                                }
                              }
                              n11041 = local read "ch2-1 transfer"() -> (w16376:bool)
                              n11042 = local read "ABORT"() -> (w16375:bool)
                              n11043 = Not(x=w16376) -> (.not. x?=w16374:bool)
                              n11044 = Compound Arithmetic op=OR(w16369, w16375, w16374) -> (w16373:bool)
                            }
                          }
                          frame #1 {
                            n11045 = while {
                              i -> [w16386]
                              stop <- w16387 stop-if-true
                              n11046 = Greater Or Equal?(x=w16386, y=100) -> (x >= y?=w16384:bool)
                              n11047 = case shown="True" w16384 {
                                frame False {
                                }
                                frame True {
                                n11048 = local write "Warning Message"("Transfer process canceled!\nCassette Servo couldn't be stopped" ("Warning Message")) -> ()
                                n11049 = local write "trns error"(TRUE ("TRNS error")) -> ()
                                }
                              }
                              n11050 = local read "Casette_Servo_Start/Stop DI"() -> (w16382:bool)
                              n11051 = case shown="True" w16382 {
                                tunnel: [TRUE ("CH1_Trns_BP_Left_DO") FALSE ("CH1_Trns_BP_Left_DO")] -> w16383
                                frame False {
                                }
                                frame True {
                                n11052 = Wait Until Next ms Multiple(millisecond multiple=u32 200) -> ()  [unwired: 1 out]
                                n11053 = local write "Casette_Servo_Start/Stop DO"(FALSE ("TRNS error")) -> ()
                                }
                              }
                              n11054 = local read "ch2-1 transfer"() -> (w16390:bool)
                              n11055 = local read "ABORT"() -> (w16389:bool)
                              n11056 = Not(x=w16390) -> (.not. x?=w16388:bool)
                              n11057 = Compound Arithmetic op=OR(w16383, w16389, w16388) -> (w16387:bool)
                            }
                          }
                          frame #2 {
                            n11058 = flat-sequence {
                              frame #0 {
                                n11059 = local write "Cassette_Servo_Speed AO"(0.0 ("Cassette_Servo_Speed AO")) -> ()
                                n11060 = Wait (ms)(milliseconds to wait=u32 100) -> ()  [unwired: 1 out]
                              }
                              frame #1 {
                                n11061 = local write "Cassette_Servo_Speed Set"(TRUE ("Cassette_Servo_Speed Set")) -> ()
                              }
                            }
                          }
                        }
                      }
                      frame True {
                      }
                    }
                  }
                }
              }
              frame #37 {
                n11062 = local read "ch2-1 transfer"() -> (w16400:bool)
                n11063 = case shown="True" w16400 {
                  frame False {
                  }
                  frame True {
                    n11064 = local read "ABORT"() -> (w16401:bool)
                    n11065 = case shown="False" w16401 {
                      frame False {
                        n11066 = local write "trns 2-1 led 17"(TRUE ("trns 1-2 led 1")) -> ()
                        n11067 = Wait (ms)(milliseconds to wait=u32 100) -> ()  [unwired: 1 out]
                      }
                      frame True {
                      }
                    }
                  }
                }
              }
              frame #38 {
                n11068 = local read "ch2-1 transfer"() -> (w16404:bool)
                n11069 = case shown="True" w16404 {
                  frame False {
                  }
                  frame True {
                    n11070 = local read "ABORT"() -> (w16405:bool)
                    n11071 = case shown="False" w16405 {
                      frame False {
                        n11072 = local read "target chamber"() -> (w16406:dbl)
                        n11073 = Equal?(x=w16406, y=1.0) -> (x = y?=w16407:bool)
                        n11074 = case shown="True" w16407 {
                          frame False {
                          }
                          frame True {
                            n11075 = while {
                              i -> [w16413]
                              stop <- w16414 stop-if-true
                              n11076 = Greater Or Equal?(x=w16413, y=100) -> (x >= y?=w16411:bool)
                              n11077 = case shown="True" w16411 {
                                frame False {
                                }
                                frame True {
                                n11078 = local write "Warning Message"("Transfer process canceled!\nCH1 Cassette Fix couldn't reached  to down position" ("Warning Message")) -> ()
                                n11079 = local write "trns error"(TRUE ("TRNS error")) -> ()
                                }
                              }
                              n11080 = local read "CH1_Cst_Fix_Down_DI"() -> (w16409:bool)
                              n11081 = case shown="False" w16409 {
                                tunnel: [FALSE ("CH1_Trns_BP_Left_DO") TRUE ("CH1_Trns_BP_Left_DO")] -> w16410
                                frame False {
                                n11082 = Wait Until Next ms Multiple(millisecond multiple=u32 200) -> ()  [unwired: 1 out]
                                n11083 = local write "CH1_Cst_Fix_DO"(TRUE ("TRNS error")) -> ()
                                }
                                frame True {
                                }
                              }
                              n11084 = local read "ch2-1 transfer"() -> (w16417:bool)
                              n11085 = local read "ABORT"() -> (w16416:bool)
                              n11086 = Not(x=w16417) -> (.not. x?=w16415:bool)
                              n11087 = Compound Arithmetic op=OR(w16410, w16416, w16415) -> (w16414:bool)
                            }
                          }